vi "run_pharmaBotExp_v1.000.vi"(0 "data in":T12={"daq_ao 1"="Dev1/ao0", "daq_ai 1"="Dev1/ai0", "experiment day folder"=path "C:/multiBot/data/debug/testing", "Multiclamp init error"=0, "Multiclamp Handle Out"=10225184, "sampling rate (Hz)"=20000, "trial name"="t1"}, 1 "auto run?":bool, 3 "which manipulator":T13(ring), 4 "HEK/slice options":enum16{"slice", "HEK"}(ring), 5 "error in":errorcluster, 6 "Validate after Experiment":bool, 7 "common cluster":T9, 11 "individual controls in":T8, 13 "images":T3={"slice image"="remote image 00000000137F745C", "pipette template"="remote image 00000000137F7D5C", "found pipette"=refnum, "pipette mask for cell tracker"=refnum, "cell images ref"=refnum}) -> (10 "Cell Looks Good?":bool=TRUE, 12 "ValidationOutputCluster":T5(array[cluster]), 14 "ValidationResults":waveform(dbl)[][](array[waveform]), 15 "ValidationPos1":T6(array[ring]), 16 "Exp. Terminated":bool, 17 "ValidationPos2":T6(array[ring]), 18 "ValidationWaveform":waveform(dbl)[](array[waveform]), 19 "error out":errorcluster)   [LabVIEW 2019] (continued)
  in  "Gap Free Iclamp G":T33={"Which Position to use for Experiment"=enum."Don't Move", "Duration (s)"=10.0, "Valve 1 Position"=2, "Valve 2 Position"=2, "Replicates"=5.0, "Iholding (pA)"=200.0, "Valve 3 Position"=2, "valve 1 used now?"=TRUE, "valve 2 used now?"=FALSE, "valve 3 used now? "=FALSE, "Record During Solution Change?"=FALSE} {"Valve 3 Position" min=1 max=8; "Iholding (pA)" step=0.1; "Replicates" min=1.0 step=1.0; "Valve 2 Position" min=1 max=8; "Valve 1 Position" min=1 max=8; "Duration (s)" min=0.0 step=0.1}
  in  "PhaseH Experiment Option":string(combo)="Single Jump"
  in  "Experiment Selection H":T20(tab)
  in  "Single Jump H":T21={"Which Position to use for Experiment"=enum."Jumper Position B-A", "Start Position (N)"="Jumper Posistion B", "Jump Position (m)"="Jumper Posistion A", "Duration (s)"=5.0, "Delay (s)"=1.0, "Pulse Width (s)"=1.0, "Valve 1 Position"=2, "Valve 2 Position"=2, "Replicates"=1.0, "Vholding (mV)"=-60.0, "Valve 3 Position"=2, "valve 1 used now?"=TRUE, "valve 2 used now?"=FALSE, "valve 3 used now? "=FALSE, "protocol Preview"=[]} {"Valve 3 Position" min=1 max=8; "Vholding (mV)" step=0.1; "Replicates" min=1.0 step=1.0; "Valve 2 Position" min=1 max=8; "Valve 1 Position" min=1 max=8; "Pulse Width (s)" min=0.0 step=0.1; "Delay (s)" min=0.0 step=0.1; "Duration (s)" min=0.0 step=0.1}
  in  "Solution Change H":T22={"Which Position to use for Experiment"=enum."Jumper Safe Position", "Duration (s)"=60.0, "Delay (s)"=1.0, "Pulse Width (s)"=30.0, "Which Valve to Change?"=1, "Valve Jump Position"=3, "Replicates"=1.0, "Vholding (mV)"=-70.0, "valve 1 used now?"=TRUE, "valve 2 used now?"=FALSE, "valve 3 used now? "=FALSE, "Valve 1 Position"=2, "Valve 2 Position"=2, "Valve 3 Position"=2, "protocol Preview"=[]} {"Valve 3 Position" min=1 max=8; "Valve 2 Position" min=1 max=8; "Valve 1 Position" min=1 max=8; "Vholding (mV)" step=0.1; "Replicates" min=1.0 step=1.0; "Valve Jump Position" min=1 max=8 step=1; "Which Valve to Change?" min=1 max=8 step=1; "Pulse Width (s)" min=0.0 step=0.1; "Delay (s)" min=0.0 step=0.1; "Duration (s)" min=0.0 step=0.1}
  in  "Voltage Step H":T23={"Which Position to use for Experiment"=enum."Jumper Safe Position", "Duration (s)"=10.0, "Delay (s)"=1.0, "Step Width (s)"=0.1, "Voltage Start (mV)"=-60.0, "Voltage Step (mV)"=0.0, "Replicates"=1.0, "Voltage End (mV)"=40.0, "Number of Step"=20.0, "Vholding (mV)"=-60.0, "Valve 1 Position"=2, "Valve 2 Position"=2, "Valve 3 Position"=2, "valve 1 used now?"=TRUE, "valve 2 used now?"=FALSE, "valve 3 used now? "=FALSE, "Total Step Time (s)"=0.0, "Maintain Final Voltage until end?"=TRUE, "protocol Preview"=[]} {"Total Step Time (s)" min=0.0 step=0.1; "Valve 3 Position" min=1 max=8; "Valve 2 Position" min=1 max=8; "Valve 1 Position" min=1 max=8; "Vholding (mV)" step=0.1; "Number of Step" min=0.0 step=1.0; "Voltage End (mV)" step=0.1; "Replicates" min=1.0 step=1.0; "Voltage Step (mV)" step=0.1; "Voltage Start (mV)" step=0.1; "Step Width (s)" step=0.1; "Delay (s)" min=0.0 step=0.1; "Duration (s)" min=0.0 step=0.1}
  in  "Voltage Ramp H":T24={"Which Position to use for Experiment"=enum."Jumper Safe Position", "Duration (s)"=10.0, "Delay (s)"=1.0, "Ramp Slope (mV/s)"=0.0, "Voltage Start (mV)"=-60.0, "Replicates"=1.0, "Voltage End (mV)"=40.0, "Ramp Duration (s)"=5.0, "Vholding (mV)"=-60.0, "Valve 1 Position"=2, "Valve 2 Position"=2, "Valve 3 Position"=2, "valve 1 used now?"=TRUE, "valve 2 used now?"=FALSE, "valve 3 used now? "=FALSE, "Maintain Final Voltage until end?"=TRUE, "protocol Preview"=[]} {"Valve 3 Position" min=1 max=8; "Valve 2 Position" min=1 max=8; "Valve 1 Position" min=1 max=8; "Ramp Duration (s)" min=0.0 step=0.1; "Voltage End (mV)" step=0.1; "Replicates" min=1.0 step=1.0; "Voltage Start (mV)" step=0.1; "Ramp Slope (mV/s)" step=0.1; "Delay (s)" min=0.0 step=0.1; "Duration (s)" min=0.0 step=0.1}
  in  "Voltage Pulse H":T25={"Which Position to use for Experiment"=enum."Jumper Safe Position", "Duration (s)"=1.0, "Delay (s)"=0.2, "Pulse 2 (s)"=0.4, "Pulse 1 (mV)"=-80.0, "Replicates"=1.0, "Pulse 1 (s)"=0.2, "Pulse 2 (mV)"=-80.0, "Vholding (mV)"=-60.0, "Valve 1 Position"=2, "Valve 2 Position"=2, "Valve 3 Position"=2, "valve 1 used now?"=TRUE, "valve 2 used now?"=FALSE, "valve 3 used now? "=FALSE, "Maintain Final Voltage until end?"=TRUE, "delta Pulse 1 (mV)"=0.0, "delta Pulse 2 (mV)"=5.0, "Sweeps"=24.0, "Final Pulse 1 (mV)"=0.0, "Final Pulse 2 (mV)"=0.0, "protocol Preview"=[]} {"Final Pulse 2 (mV)" step=0.1; "Final Pulse 1 (mV)" step=0.1; "Sweeps" min=1.0 step=1.0; "delta Pulse 2 (mV)" step=0.1; "delta Pulse 1 (mV)" step=0.1; "Valve 3 Position" min=1 max=8; "Valve 2 Position" min=1 max=8; "Valve 1 Position" min=1 max=8; "Vholding (mV)" step=0.1; "Pulse 2 (mV)" step=0.1; "Pulse 1 (s)" min=0.0 step=0.1; "Replicates" min=1.0 step=1.0; "Pulse 1 (mV)" step=0.1; "Pulse 2 (s)" min=0.0 step=0.1; "Delay (s)" min=0.0 step=0.1; "Duration (s)" min=0.0 step=0.1}
  in  "Jump Train H":T26={"Which Position to use for Experiment"=enum."Jumper Safe Position", "Start Position (N)"="", "Jump Position (m)"="", "Duration (s)"=20.0, "Delay (s)"=1.0, "Pulse Width (s)"=1.0, "Valve 1 Position"=1, "Valve 2 Position"=1, "Replicates"=1.0, "Pulse Period (s)"=2.0, "Vholding (mV)"=-60.0, "Number of Pulses"=5.0, "valve 1 used now?"=TRUE, "valve 2 used now?"=FALSE, "valve 3 used now? "=FALSE, "Valve 3 Position"=1, "protocol Preview"=[]} {"Valve 3 Position" min=1 max=8; "Number of Pulses" min=0.0 step=1.0; "Vholding (mV)" step=0.1; "Pulse Period (s)" min=0.0 step=0.1; "Replicates" min=1.0 step=1.0; "Valve 2 Position" min=1 max=8; "Valve 1 Position" min=1 max=8; "Pulse Width (s)" min=0.0 step=0.1; "Delay (s)" min=0.0 step=0.1; "Duration (s)" min=0.0 step=0.1}
  in  "Paired Pulse H":T27={"Which Position to use for Experiment"=enum."Jumper Safe Position", "Start Position (N)"="", "Jump Position (m)"="", "Duration (s)"=10.0, "Delay (s)"=1.0, "Pulse Width (s)"=1.0, "Replicates"=1.0, "Pulse Delay (s)"=1.0, "Pulse Delta Delay (s)"=0.5, "Vholding (mV)"=-60.0, "Valve 1 Position"=1, "Valve 2 Position"=1, "valve 1 used now?"=TRUE, "valve 2 used now?"=FALSE, "valve 3 used now? "=FALSE, "Valve 3 Position"=1, "protocol Preview"=[]} {"Valve 3 Position" min=1 max=8; "Valve 2 Position" min=1 max=8; "Valve 1 Position" min=1 max=8; "Vholding (mV)" step=0.1; "Pulse Delta Delay (s)" min=0.0 step=0.1; "Pulse Delay (s)" min=0.0 step=0.1; "Replicates" min=1.0 step=1.0; "Pulse Width (s)" min=0.0 step=0.1; "Delay (s)" min=0.0 step=0.1; "Duration (s)" min=0.0 step=0.1}
  in  "Single Manip Jump H":T28={"Start Position (N)"=enum."Jumper Position B", "Duration (s)"=8.0, "Delay (s)"=0.5, "Pulse Width (s)"=1.0, "Valve 1 Position"=2, "Valve 2 Position"=2, "Replicates"=10.0, "Jump Position (m)"=enum."Jumper Position A", "Vholding (mV)"=-60.0, "Valve 3 Position"=2, "valve 1 used now?"=TRUE, "valve 2 used now?"=FALSE, "valve 3 used now? "=FALSE, "protocol Preview"=[]} {"Valve 3 Position" min=1 max=8; "Vholding (mV)" step=0.1; "Replicates" min=1.0 step=1.0; "Valve 2 Position" min=1 max=8; "Valve 1 Position" min=1 max=8; "Pulse Width (s)" min=0.0 step=0.1; "Delay (s)" min=0.0 step=0.1; "Duration (s)" min=0.0 step=0.1}
  in  "Gap Free H":T29={"Which Position to use for Experiment"=enum."Don't Move", "Duration (s)"=120.0, "Valve 1 Position"=1, "Valve 2 Position"=1, "Replicates"=2.0, "Vholding (mV)"=-60.0, "Valve 3 Position"=1, "valve 1 used now?"=TRUE, "valve 2 used now?"=FALSE, "valve 3 used now? "=FALSE, "Record During Solution Change?"=TRUE} {"Valve 3 Position" min=1 max=8; "Vholding (mV)" step=0.1; "Replicates" min=1.0 step=1.0; "Valve 2 Position" min=1 max=8; "Valve 1 Position" min=1 max=8; "Duration (s)" min=0.0 step=0.1}
  in  "Multi Manip Jump H":T30={"Start Position (N)"=enum."Jumper Position C", "Duration (s)"=20.0, "Delay (s)"=2.0, "Valve 1 Position"=2, "Valve 2 Position"=2, "Replicates"=5.0, "Vholding (mV)"=-60.0, "Valve 3 Position"=2, "valve 1 used now?"=TRUE, "valve 2 used now?"=FALSE, "valve 3 used now? "=FALSE, "Jump Position Array"=[enum."Jumper Position B", enum."Jumper Position A", enum."Jumper Position B", enum."Jumper Position C"], "Position Dwell Time (s)"=[2.0, 4.0, 4.0, 4.0], "protocol Preview"=[]} {"Position Dwell Time (s)" min=0.0 step=0.1; "Vholding (mV)" step=0.1; "Replicates" min=1.0 step=1.0; "Valve 2 Position" min=1 max=8; "Delay (s)" min=0.0 step=0.1; "Duration (s)" min=0.0 step=0.1}
  in  "Current Pulse H":T31={"Which Position to use for Experiment"=enum."Jumper Safe Position", "Duration (s)"=1.0, "Delay (s)"=0.2, "Pulse 2 (s)"=0.4, "Pulse 1 (pA)"=-400.0, "Replicates"=1.0, "Pulse 1 (s)"=0.6, "Pulse 2 (pA)"=-80.0, "Iholding (pA)"=0.0, "Valve 1 Position"=2, "Valve 2 Position"=2, "Valve 3 Position"=2, "valve 1 used now?"=TRUE, "valve 2 used now?"=FALSE, "valve 3 used now? "=FALSE, "Maintain Final Voltage until end?"=FALSE, "delta Pulse 1 (pA)"=50.0, "delta Pulse 2 (pA)"=5.0, "Sweeps"=24.0, "Final Pulse 1 (pA)"=0.0, "Final Pulse 2 (pA)"=0.0, "protocol Preview"=[]} {"Final Pulse 2 (pA)" step=0.1; "Final Pulse 1 (pA)" step=0.1; "Sweeps" min=1.0 step=1.0; "delta Pulse 2 (pA)" step=0.1; "delta Pulse 1 (pA)" step=0.1; "Valve 3 Position" min=1 max=8; "Valve 2 Position" min=1 max=8; "Valve 1 Position" min=1 max=8; "Iholding (pA)" step=0.1; "Pulse 2 (pA)" step=0.1; "Pulse 1 (s)" min=0.0 step=0.1; "Replicates" min=1.0 step=1.0; "Pulse 1 (pA)" step=0.1; "Pulse 2 (s)" min=0.0 step=0.1; "Delay (s)" min=0.0 step=0.1; "Duration (s)" min=0.0 step=0.1}
  in  "Current Ramp H":T32={"Which Position to use for Experiment"=enum."Jumper Safe Position", "Duration (s)"=10.0, "Delay (s)"=1.0, "Ramp Slope (pA/s)"=0.0, "Current Start (pA)"=-200.0, "Replicates"=1.0, "Current End (pA)"=500.0, "Ramp Duration (s)"=5.0, "Iholding (pA)"=0.0, "Valve 1 Position"=2, "Valve 2 Position"=2, "Valve 3 Position"=2, "valve 1 used now?"=TRUE, "valve 2 used now?"=FALSE, "valve 3 used now? "=FALSE, "Maintain Final Voltage until end?"=FALSE, "protocol Preview"=[]} {"Valve 3 Position" min=1 max=8; "Valve 2 Position" min=1 max=8; "Valve 1 Position" min=1 max=8; "Ramp Duration (s)" min=0.0 step=0.1; "Current End (pA)" step=0.1; "Replicates" min=1.0 step=1.0; "Current Start (pA)" step=0.1; "Ramp Slope (pA/s)" step=0.1; "Delay (s)" min=0.0 step=0.1; "Duration (s)" min=0.0 step=0.1}
  in  "Gap Free Iclamp H":T33={"Which Position to use for Experiment"=enum."Don't Move", "Duration (s)"=10.0, "Valve 1 Position"=2, "Valve 2 Position"=2, "Replicates"=5.0, "Iholding (pA)"=200.0, "Valve 3 Position"=2, "valve 1 used now?"=TRUE, "valve 2 used now?"=FALSE, "valve 3 used now? "=FALSE, "Record During Solution Change?"=FALSE} {"Valve 3 Position" min=1 max=8; "Iholding (pA)" step=0.1; "Replicates" min=1.0 step=1.0; "Valve 2 Position" min=1 max=8; "Valve 1 Position" min=1 max=8; "Duration (s)" min=0.0 step=0.1}
  in  "PhaseI Experiment Option":string(combo)="Single Manip Jump"
  in  "Experiment Selection I":T20(tab)=enum."Single Manip Jump"
  in  "Single Jump I":T21={"Which Position to use for Experiment"=enum."Jumper Position B-A", "Start Position (N)"="Jumper Posistion B", "Jump Position (m)"="Jumper Posistion A", "Duration (s)"=5.0, "Delay (s)"=1.0, "Pulse Width (s)"=1.0, "Valve 1 Position"=2, "Valve 2 Position"=2, "Replicates"=10.0, "Vholding (mV)"=-60.0, "Valve 3 Position"=2, "valve 1 used now?"=TRUE, "valve 2 used now?"=FALSE, "valve 3 used now? "=FALSE, "protocol Preview"=[]} {"Valve 3 Position" min=1 max=8; "Vholding (mV)" step=0.1; "Replicates" min=1.0 step=1.0; "Valve 2 Position" min=1 max=8; "Valve 1 Position" min=1 max=8; "Pulse Width (s)" min=0.0 step=0.1; "Delay (s)" min=0.0 step=0.1; "Duration (s)" min=0.0 step=0.1}
  in  "Solution Change I":T22={"Which Position to use for Experiment"=enum."Jumper Safe Position", "Duration (s)"=60.0, "Delay (s)"=1.0, "Pulse Width (s)"=30.0, "Which Valve to Change?"=1, "Valve Jump Position"=3, "Replicates"=1.0, "Vholding (mV)"=-70.0, "valve 1 used now?"=TRUE, "valve 2 used now?"=FALSE, "valve 3 used now? "=FALSE, "Valve 1 Position"=2, "Valve 2 Position"=2, "Valve 3 Position"=2, "protocol Preview"=[]} {"Valve 3 Position" min=1 max=8; "Valve 2 Position" min=1 max=8; "Valve 1 Position" min=1 max=8; "Vholding (mV)" step=0.1; "Replicates" min=1.0 step=1.0; "Valve Jump Position" min=1 max=8 step=1; "Which Valve to Change?" min=1 max=8 step=1; "Pulse Width (s)" min=0.0 step=0.1; "Delay (s)" min=0.0 step=0.1; "Duration (s)" min=0.0 step=0.1}
  in  "Voltage Step I":T23={"Which Position to use for Experiment"=enum."Jumper Safe Position", "Duration (s)"=10.0, "Delay (s)"=1.0, "Step Width (s)"=0.1, "Voltage Start (mV)"=-60.0, "Voltage Step (mV)"=0.0, "Replicates"=1.0, "Voltage End (mV)"=40.0, "Number of Step"=20.0, "Vholding (mV)"=-60.0, "Valve 1 Position"=2, "Valve 2 Position"=2, "Valve 3 Position"=2, "valve 1 used now?"=TRUE, "valve 2 used now?"=FALSE, "valve 3 used now? "=FALSE, "Total Step Time (s)"=0.0, "Maintain Final Voltage until end?"=TRUE, "protocol Preview"=[]} {"Total Step Time (s)" min=0.0 step=0.1; "Valve 3 Position" min=1 max=8; "Valve 2 Position" min=1 max=8; "Valve 1 Position" min=1 max=8; "Vholding (mV)" step=0.1; "Number of Step" min=0.0 step=1.0; "Voltage End (mV)" step=0.1; "Replicates" min=1.0 step=1.0; "Voltage Step (mV)" step=0.1; "Voltage Start (mV)" step=0.1; "Step Width (s)" step=0.1; "Delay (s)" min=0.0 step=0.1; "Duration (s)" min=0.0 step=0.1}
  in  "Voltage Ramp I":T24={"Which Position to use for Experiment"=enum."Jumper Safe Position", "Duration (s)"=10.0, "Delay (s)"=1.0, "Ramp Slope (mV/s)"=0.0, "Voltage Start (mV)"=-60.0, "Replicates"=1.0, "Voltage End (mV)"=40.0, "Ramp Duration (s)"=5.0, "Vholding (mV)"=-60.0, "Valve 1 Position"=2, "Valve 2 Position"=2, "Valve 3 Position"=2, "valve 1 used now?"=TRUE, "valve 2 used now?"=FALSE, "valve 3 used now? "=FALSE, "Maintain Final Voltage until end?"=TRUE, "protocol Preview"=[]} {"Valve 3 Position" min=1 max=8; "Valve 2 Position" min=1 max=8; "Valve 1 Position" min=1 max=8; "Ramp Duration (s)" min=0.0 step=0.1; "Voltage End (mV)" step=0.1; "Replicates" min=1.0 step=1.0; "Voltage Start (mV)" step=0.1; "Ramp Slope (mV/s)" step=0.1; "Delay (s)" min=0.0 step=0.1; "Duration (s)" min=0.0 step=0.1}
  in  "Voltage Pulse I":T25={"Which Position to use for Experiment"=enum."Jumper Safe Position", "Duration (s)"=1.0, "Delay (s)"=0.2, "Pulse 2 (s)"=0.4, "Pulse 1 (mV)"=-80.0, "Replicates"=1.0, "Pulse 1 (s)"=0.2, "Pulse 2 (mV)"=-80.0, "Vholding (mV)"=-60.0, "Valve 1 Position"=2, "Valve 2 Position"=2, "Valve 3 Position"=2, "valve 1 used now?"=TRUE, "valve 2 used now?"=FALSE, "valve 3 used now? "=FALSE, "Maintain Final Voltage until end?"=TRUE, "delta Pulse 1 (mV)"=0.0, "delta Pulse 2 (mV)"=5.0, "Sweeps"=24.0, "Final Pulse 1 (mV)"=0.0, "Final Pulse 2 (mV)"=0.0, "protocol Preview"=[]} {"Final Pulse 2 (mV)" step=0.1; "Final Pulse 1 (mV)" step=0.1; "Sweeps" min=1.0 step=1.0; "delta Pulse 2 (mV)" step=0.1; "delta Pulse 1 (mV)" step=0.1; "Valve 3 Position" min=1 max=8; "Valve 2 Position" min=1 max=8; "Valve 1 Position" min=1 max=8; "Vholding (mV)" step=0.1; "Pulse 2 (mV)" step=0.1; "Pulse 1 (s)" min=0.0 step=0.1; "Replicates" min=1.0 step=1.0; "Pulse 1 (mV)" step=0.1; "Pulse 2 (s)" min=0.0 step=0.1; "Delay (s)" min=0.0 step=0.1; "Duration (s)" min=0.0 step=0.1}
  in  "Jump Train I":T26={"Which Position to use for Experiment"=enum."Jumper Safe Position", "Start Position (N)"="", "Jump Position (m)"="", "Duration (s)"=20.0, "Delay (s)"=1.0, "Pulse Width (s)"=1.0, "Valve 1 Position"=1, "Valve 2 Position"=1, "Replicates"=1.0, "Pulse Period (s)"=2.0, "Vholding (mV)"=-60.0, "Number of Pulses"=5.0, "valve 1 used now?"=TRUE, "valve 2 used now?"=FALSE, "valve 3 used now? "=FALSE, "Valve 3 Position"=1, "protocol Preview"=[]} {"Valve 3 Position" min=1 max=8; "Number of Pulses" min=0.0 step=1.0; "Vholding (mV)" step=0.1; "Pulse Period (s)" min=0.0 step=0.1; "Replicates" min=1.0 step=1.0; "Valve 2 Position" min=1 max=8; "Valve 1 Position" min=1 max=8; "Pulse Width (s)" min=0.0 step=0.1; "Delay (s)" min=0.0 step=0.1; "Duration (s)" min=0.0 step=0.1}
  in  "Paired Pulse I":T27={"Which Position to use for Experiment"=enum."Jumper Safe Position", "Start Position (N)"="", "Jump Position (m)"="", "Duration (s)"=10.0, "Delay (s)"=1.0, "Pulse Width (s)"=1.0, "Replicates"=1.0, "Pulse Delay (s)"=1.0, "Pulse Delta Delay (s)"=0.5, "Vholding (mV)"=-60.0, "Valve 1 Position"=1, "Valve 2 Position"=1, "valve 1 used now?"=TRUE, "valve 2 used now?"=FALSE, "valve 3 used now? "=FALSE, "Valve 3 Position"=1, "protocol Preview"=[]} {"Valve 3 Position" min=1 max=8; "Valve 2 Position" min=1 max=8; "Valve 1 Position" min=1 max=8; "Vholding (mV)" step=0.1; "Pulse Delta Delay (s)" min=0.0 step=0.1; "Pulse Delay (s)" min=0.0 step=0.1; "Replicates" min=1.0 step=1.0; "Pulse Width (s)" min=0.0 step=0.1; "Delay (s)" min=0.0 step=0.1; "Duration (s)" min=0.0 step=0.1}
  in  "Single Manip Jump I":T28={"Start Position (N)"=enum."Jumper Position B", "Duration (s)"=8.0, "Delay (s)"=0.5, "Pulse Width (s)"=1.0, "Valve 1 Position"=2, "Valve 2 Position"=2, "Replicates"=1.0, "Jump Position (m)"=enum."Jumper Position A", "Vholding (mV)"=-60.0, "Valve 3 Position"=2, "valve 1 used now?"=TRUE, "valve 2 used now?"=FALSE, "valve 3 used now? "=FALSE, "protocol Preview"=[]} {"Valve 3 Position" min=1 max=8; "Vholding (mV)" step=0.1; "Replicates" min=1.0 step=1.0; "Valve 2 Position" min=1 max=8; "Valve 1 Position" min=1 max=8; "Pulse Width (s)" min=0.0 step=0.1; "Delay (s)" min=0.0 step=0.1; "Duration (s)" min=0.0 step=0.1}
  in  "Gap Free I":T29={"Which Position to use for Experiment"=enum."Jumper Position B", "Duration (s)"=10.0, "Valve 1 Position"=2, "Valve 2 Position"=2, "Replicates"=5.0, "Vholding (mV)"=-60.0, "Valve 3 Position"=2, "valve 1 used now?"=TRUE, "valve 2 used now?"=FALSE, "valve 3 used now? "=FALSE, "Record During Solution Change?"=FALSE} {"Valve 3 Position" min=1 max=8; "Vholding (mV)" step=0.1; "Replicates" min=1.0 step=1.0; "Valve 2 Position" min=1 max=8; "Valve 1 Position" min=1 max=8; "Duration (s)" min=0.0 step=0.1}
  in  "Multi Manip Jump I":T30={"Start Position (N)"=enum."Jumper Position C", "Duration (s)"=20.0, "Delay (s)"=2.0, "Valve 1 Position"=2, "Valve 2 Position"=2, "Replicates"=5.0, "Vholding (mV)"=-60.0, "Valve 3 Position"=2, "valve 1 used now?"=TRUE, "valve 2 used now?"=FALSE, "valve 3 used now? "=FALSE, "Jump Position Array"=[enum."Jumper Position B", enum."Jumper Position A", enum."Jumper Position B", enum."Jumper Position C"], "Position Dwell Time (s)"=[2.0, 4.0, 4.0, 4.0], "protocol Preview"=[]} {"Position Dwell Time (s)" min=0.0 step=0.1; "Vholding (mV)" step=0.1; "Replicates" min=1.0 step=1.0; "Valve 2 Position" min=1 max=8; "Delay (s)" min=0.0 step=0.1; "Duration (s)" min=0.0 step=0.1}
  in  "Current Pulse I":T31={"Which Position to use for Experiment"=enum."Jumper Safe Position", "Duration (s)"=1.0, "Delay (s)"=0.2, "Pulse 2 (s)"=0.4, "Pulse 1 (pA)"=-400.0, "Replicates"=1.0, "Pulse 1 (s)"=0.6, "Pulse 2 (pA)"=-80.0, "Iholding (pA)"=0.0, "Valve 1 Position"=2, "Valve 2 Position"=2, "Valve 3 Position"=2, "valve 1 used now?"=TRUE, "valve 2 used now?"=FALSE, "valve 3 used now? "=FALSE, "Maintain Final Voltage until end?"=FALSE, "delta Pulse 1 (pA)"=50.0, "delta Pulse 2 (pA)"=5.0, "Sweeps"=24.0, "Final Pulse 1 (pA)"=0.0, "Final Pulse 2 (pA)"=0.0, "protocol Preview"=[]} {"Final Pulse 2 (pA)" step=0.1; "Final Pulse 1 (pA)" step=0.1; "Sweeps" min=1.0 step=1.0; "delta Pulse 2 (pA)" step=0.1; "delta Pulse 1 (pA)" step=0.1; "Valve 3 Position" min=1 max=8; "Valve 2 Position" min=1 max=8; "Valve 1 Position" min=1 max=8; "Iholding (pA)" step=0.1; "Pulse 2 (pA)" step=0.1; "Pulse 1 (s)" min=0.0 step=0.1; "Replicates" min=1.0 step=1.0; "Pulse 1 (pA)" step=0.1; "Pulse 2 (s)" min=0.0 step=0.1; "Delay (s)" min=0.0 step=0.1; "Duration (s)" min=0.0 step=0.1}
  in  "Current Ramp I":T32={"Which Position to use for Experiment"=enum."Jumper Safe Position", "Duration (s)"=10.0, "Delay (s)"=1.0, "Ramp Slope (pA/s)"=0.0, "Current Start (pA)"=-200.0, "Replicates"=1.0, "Current End (pA)"=500.0, "Ramp Duration (s)"=5.0, "Iholding (pA)"=0.0, "Valve 1 Position"=2, "Valve 2 Position"=2, "Valve 3 Position"=2, "valve 1 used now?"=TRUE, "valve 2 used now?"=FALSE, "valve 3 used now? "=FALSE, "Maintain Final Voltage until end?"=FALSE, "protocol Preview"=[]} {"Valve 3 Position" min=1 max=8; "Valve 2 Position" min=1 max=8; "Valve 1 Position" min=1 max=8; "Ramp Duration (s)" min=0.0 step=0.1; "Current End (pA)" step=0.1; "Replicates" min=1.0 step=1.0; "Current Start (pA)" step=0.1; "Ramp Slope (pA/s)" step=0.1; "Delay (s)" min=0.0 step=0.1; "Duration (s)" min=0.0 step=0.1}
  in  "Gap Free Iclamp I":T33={"Which Position to use for Experiment"=enum."Don't Move", "Duration (s)"=10.0, "Valve 1 Position"=2, "Valve 2 Position"=2, "Replicates"=5.0, "Iholding (pA)"=200.0, "Valve 3 Position"=2, "valve 1 used now?"=TRUE, "valve 2 used now?"=FALSE, "valve 3 used now? "=FALSE, "Record During Solution Change?"=FALSE} {"Valve 3 Position" min=1 max=8; "Iholding (pA)" step=0.1; "Replicates" min=1.0 step=1.0; "Valve 2 Position" min=1 max=8; "Valve 1 Position" min=1 max=8; "Duration (s)" min=0.0 step=0.1}
  in  "PhaseJ Experiment Option":string(combo)="Multi M. Jump"
  in  "Experiment Selection J":T20(tab)=enum."Multi M. Jump"
  in  "Single Jump J":T21={"Which Position to use for Experiment"=enum."Jumper Position B-A", "Start Position (N)"="Jumper Posistion B", "Jump Position (m)"="Jumper Posistion A", "Duration (s)"=5.0, "Delay (s)"=1.0, "Pulse Width (s)"=1.0, "Valve 1 Position"=2, "Valve 2 Position"=2, "Replicates"=10.0, "Vholding (mV)"=-60.0, "Valve 3 Position"=2, "valve 1 used now?"=TRUE, "valve 2 used now?"=FALSE, "valve 3 used now? "=FALSE, "protocol Preview"=[]} {"Valve 3 Position" min=1 max=8; "Vholding (mV)" step=0.1; "Replicates" min=1.0 step=1.0; "Valve 2 Position" min=1 max=8; "Valve 1 Position" min=1 max=8; "Pulse Width (s)" min=0.0 step=0.1; "Delay (s)" min=0.0 step=0.1; "Duration (s)" min=0.0 step=0.1}
  in  "Solution Change J":T22={"Which Position to use for Experiment"=enum."Jumper Safe Position", "Duration (s)"=60.0, "Delay (s)"=1.0, "Pulse Width (s)"=30.0, "Which Valve to Change?"=1, "Valve Jump Position"=3, "Replicates"=1.0, "Vholding (mV)"=-70.0, "valve 1 used now?"=TRUE, "valve 2 used now?"=FALSE, "valve 3 used now? "=FALSE, "Valve 1 Position"=2, "Valve 2 Position"=2, "Valve 3 Position"=2, "protocol Preview"=[]} {"Valve 3 Position" min=1 max=8; "Valve 2 Position" min=1 max=8; "Valve 1 Position" min=1 max=8; "Vholding (mV)" step=0.1; "Replicates" min=1.0 step=1.0; "Valve Jump Position" min=1 max=8 step=1; "Which Valve to Change?" min=1 max=8 step=1; "Pulse Width (s)" min=0.0 step=0.1; "Delay (s)" min=0.0 step=0.1; "Duration (s)" min=0.0 step=0.1}
  in  "Voltage Step J":T23={"Which Position to use for Experiment"=enum."Jumper Safe Position", "Duration (s)"=10.0, "Delay (s)"=1.0, "Step Width (s)"=0.1, "Voltage Start (mV)"=-60.0, "Voltage Step (mV)"=0.0, "Replicates"=1.0, "Voltage End (mV)"=40.0, "Number of Step"=20.0, "Vholding (mV)"=-60.0, "Valve 1 Position"=2, "Valve 2 Position"=2, "Valve 3 Position"=2, "valve 1 used now?"=TRUE, "valve 2 used now?"=FALSE, "valve 3 used now? "=FALSE, "Total Step Time (s)"=0.0, "Maintain Final Voltage until end?"=TRUE, "protocol Preview"=[]} {"Total Step Time (s)" min=0.0 step=0.1; "Valve 3 Position" min=1 max=8; "Valve 2 Position" min=1 max=8; "Valve 1 Position" min=1 max=8; "Vholding (mV)" step=0.1; "Number of Step" min=0.0 step=1.0; "Voltage End (mV)" step=0.1; "Replicates" min=1.0 step=1.0; "Voltage Step (mV)" step=0.1; "Voltage Start (mV)" step=0.1; "Step Width (s)" step=0.1; "Delay (s)" min=0.0 step=0.1; "Duration (s)" min=0.0 step=0.1}
  in  "Voltage Ramp J":T24={"Which Position to use for Experiment"=enum."Jumper Safe Position", "Duration (s)"=10.0, "Delay (s)"=1.0, "Ramp Slope (mV/s)"=0.0, "Voltage Start (mV)"=-60.0, "Replicates"=1.0, "Voltage End (mV)"=40.0, "Ramp Duration (s)"=5.0, "Vholding (mV)"=-60.0, "Valve 1 Position"=2, "Valve 2 Position"=2, "Valve 3 Position"=2, "valve 1 used now?"=TRUE, "valve 2 used now?"=FALSE, "valve 3 used now? "=FALSE, "Maintain Final Voltage until end?"=TRUE, "protocol Preview"=[]} {"Valve 3 Position" min=1 max=8; "Valve 2 Position" min=1 max=8; "Valve 1 Position" min=1 max=8; "Ramp Duration (s)" min=0.0 step=0.1; "Voltage End (mV)" step=0.1; "Replicates" min=1.0 step=1.0; "Voltage Start (mV)" step=0.1; "Ramp Slope (mV/s)" step=0.1; "Delay (s)" min=0.0 step=0.1; "Duration (s)" min=0.0 step=0.1}
  in  "Voltage Pulse J":T25={"Which Position to use for Experiment"=enum."Jumper Safe Position", "Duration (s)"=1.0, "Delay (s)"=0.2, "Pulse 2 (s)"=0.4, "Pulse 1 (mV)"=-80.0, "Replicates"=1.0, "Pulse 1 (s)"=0.2, "Pulse 2 (mV)"=-80.0, "Vholding (mV)"=-60.0, "Valve 1 Position"=2, "Valve 2 Position"=2, "Valve 3 Position"=2, "valve 1 used now?"=TRUE, "valve 2 used now?"=FALSE, "valve 3 used now? "=FALSE, "Maintain Final Voltage until end?"=TRUE, "delta Pulse 1 (mV)"=0.0, "delta Pulse 2 (mV)"=5.0, "Sweeps"=24.0, "Final Pulse 1 (mV)"=0.0, "Final Pulse 2 (mV)"=0.0, "protocol Preview"=[]} {"Final Pulse 2 (mV)" step=0.1; "Final Pulse 1 (mV)" step=0.1; "Sweeps" min=1.0 step=1.0; "delta Pulse 2 (mV)" step=0.1; "delta Pulse 1 (mV)" step=0.1; "Valve 3 Position" min=1 max=8; "Valve 2 Position" min=1 max=8; "Valve 1 Position" min=1 max=8; "Vholding (mV)" step=0.1; "Pulse 2 (mV)" step=0.1; "Pulse 1 (s)" min=0.0 step=0.1; "Replicates" min=1.0 step=1.0; "Pulse 1 (mV)" step=0.1; "Pulse 2 (s)" min=0.0 step=0.1; "Delay (s)" min=0.0 step=0.1; "Duration (s)" min=0.0 step=0.1}
  in  "Jump Train J":T26={"Which Position to use for Experiment"=enum."Jumper Safe Position", "Start Position (N)"="", "Jump Position (m)"="", "Duration (s)"=20.0, "Delay (s)"=1.0, "Pulse Width (s)"=1.0, "Valve 1 Position"=1, "Valve 2 Position"=1, "Replicates"=1.0, "Pulse Period (s)"=2.0, "Vholding (mV)"=-60.0, "Number of Pulses"=5.0, "valve 1 used now?"=TRUE, "valve 2 used now?"=FALSE, "valve 3 used now? "=FALSE, "Valve 3 Position"=1, "protocol Preview"=[]} {"Valve 3 Position" min=1 max=8; "Number of Pulses" min=0.0 step=1.0; "Vholding (mV)" step=0.1; "Pulse Period (s)" min=0.0 step=0.1; "Replicates" min=1.0 step=1.0; "Valve 2 Position" min=1 max=8; "Valve 1 Position" min=1 max=8; "Pulse Width (s)" min=0.0 step=0.1; "Delay (s)" min=0.0 step=0.1; "Duration (s)" min=0.0 step=0.1}
  in  "Paired Pulse J":T27={"Which Position to use for Experiment"=enum."Jumper Safe Position", "Start Position (N)"="", "Jump Position (m)"="", "Duration (s)"=10.0, "Delay (s)"=1.0, "Pulse Width (s)"=1.0, "Replicates"=1.0, "Pulse Delay (s)"=1.0, "Pulse Delta Delay (s)"=0.5, "Vholding (mV)"=-60.0, "Valve 1 Position"=1, "Valve 2 Position"=1, "valve 1 used now?"=TRUE, "valve 2 used now?"=FALSE, "valve 3 used now? "=FALSE, "Valve 3 Position"=1, "protocol Preview"=[]} {"Valve 3 Position" min=1 max=8; "Valve 2 Position" min=1 max=8; "Valve 1 Position" min=1 max=8; "Vholding (mV)" step=0.1; "Pulse Delta Delay (s)" min=0.0 step=0.1; "Pulse Delay (s)" min=0.0 step=0.1; "Replicates" min=1.0 step=1.0; "Pulse Width (s)" min=0.0 step=0.1; "Delay (s)" min=0.0 step=0.1; "Duration (s)" min=0.0 step=0.1}
  in  "Single Manip Jump J":T28={"Start Position (N)"=enum."Jumper Position B", "Duration (s)"=8.0, "Delay (s)"=0.5, "Pulse Width (s)"=1.0, "Valve 1 Position"=2, "Valve 2 Position"=2, "Replicates"=10.0, "Jump Position (m)"=enum."Jumper Position A", "Vholding (mV)"=-60.0, "Valve 3 Position"=2, "valve 1 used now?"=TRUE, "valve 2 used now?"=FALSE, "valve 3 used now? "=FALSE, "protocol Preview"=[]} {"Valve 3 Position" min=1 max=8; "Vholding (mV)" step=0.1; "Replicates" min=1.0 step=1.0; "Valve 2 Position" min=1 max=8; "Valve 1 Position" min=1 max=8; "Pulse Width (s)" min=0.0 step=0.1; "Delay (s)" min=0.0 step=0.1; "Duration (s)" min=0.0 step=0.1}
  in  "Gap Free J":T29={"Which Position to use for Experiment"=enum."Jumper Position B", "Duration (s)"=10.0, "Valve 1 Position"=2, "Valve 2 Position"=2, "Replicates"=5.0, "Vholding (mV)"=-60.0, "Valve 3 Position"=2, "valve 1 used now?"=TRUE, "valve 2 used now?"=FALSE, "valve 3 used now? "=FALSE, "Record During Solution Change?"=FALSE} {"Valve 3 Position" min=1 max=8; "Vholding (mV)" step=0.1; "Replicates" min=1.0 step=1.0; "Valve 2 Position" min=1 max=8; "Valve 1 Position" min=1 max=8; "Duration (s)" min=0.0 step=0.1}
  in  "Multi Manip Jump J":T30={"Start Position (N)"=enum."Jumper Position C", "Duration (s)"=20.0, "Delay (s)"=2.0, "Valve 1 Position"=2, "Valve 2 Position"=2, "Replicates"=1.0, "Vholding (mV)"=-60.0, "Valve 3 Position"=2, "valve 1 used now?"=TRUE, "valve 2 used now?"=FALSE, "valve 3 used now? "=FALSE, "Jump Position Array"=[enum."Jumper Position B", enum."Jumper Position A", enum."Jumper Position B", enum."Jumper Position C"], "Position Dwell Time (s)"=[2.0, 4.0, 4.0, 4.0], "protocol Preview"=[]} {"Position Dwell Time (s)" min=0.0 step=0.1; "Vholding (mV)" step=0.1; "Replicates" min=1.0 step=1.0; "Valve 2 Position" min=1 max=8; "Delay (s)" min=0.0 step=0.1; "Duration (s)" min=0.0 step=0.1}
  in  "Current Pulse J":T31={"Which Position to use for Experiment"=enum."Jumper Safe Position", "Duration (s)"=1.0, "Delay (s)"=0.2, "Pulse 2 (s)"=0.4, "Pulse 1 (pA)"=-400.0, "Replicates"=1.0, "Pulse 1 (s)"=0.6, "Pulse 2 (pA)"=-80.0, "Iholding (pA)"=0.0, "Valve 1 Position"=2, "Valve 2 Position"=2, "Valve 3 Position"=2, "valve 1 used now?"=TRUE, "valve 2 used now?"=FALSE, "valve 3 used now? "=FALSE, "Maintain Final Voltage until end?"=FALSE, "delta Pulse 1 (pA)"=50.0, "delta Pulse 2 (pA)"=5.0, "Sweeps"=24.0, "Final Pulse 1 (pA)"=0.0, "Final Pulse 2 (pA)"=0.0, "protocol Preview"=[]} {"Final Pulse 2 (pA)" step=0.1; "Final Pulse 1 (pA)" step=0.1; "Sweeps" min=1.0 step=1.0; "delta Pulse 2 (pA)" step=0.1; "delta Pulse 1 (pA)" step=0.1; "Valve 3 Position" min=1 max=8; "Valve 2 Position" min=1 max=8; "Valve 1 Position" min=1 max=8; "Iholding (pA)" step=0.1; "Pulse 2 (pA)" step=0.1; "Pulse 1 (s)" min=0.0 step=0.1; "Replicates" min=1.0 step=1.0; "Pulse 1 (pA)" step=0.1; "Pulse 2 (s)" min=0.0 step=0.1; "Delay (s)" min=0.0 step=0.1; "Duration (s)" min=0.0 step=0.1}
  in  "Current Ramp J":T32={"Which Position to use for Experiment"=enum."Jumper Safe Position", "Duration (s)"=10.0, "Delay (s)"=1.0, "Ramp Slope (pA/s)"=0.0, "Current Start (pA)"=-200.0, "Replicates"=1.0, "Current End (pA)"=500.0, "Ramp Duration (s)"=5.0, "Iholding (pA)"=0.0, "Valve 1 Position"=2, "Valve 2 Position"=2, "Valve 3 Position"=2, "valve 1 used now?"=TRUE, "valve 2 used now?"=FALSE, "valve 3 used now? "=FALSE, "Maintain Final Voltage until end?"=FALSE, "protocol Preview"=[]} {"Valve 3 Position" min=1 max=8; "Valve 2 Position" min=1 max=8; "Valve 1 Position" min=1 max=8; "Ramp Duration (s)" min=0.0 step=0.1; "Current End (pA)" step=0.1; "Replicates" min=1.0 step=1.0; "Current Start (pA)" step=0.1; "Ramp Slope (pA/s)" step=0.1; "Delay (s)" min=0.0 step=0.1; "Duration (s)" min=0.0 step=0.1}
  in  "Gap Free Iclamp J":T33={"Which Position to use for Experiment"=enum."Don't Move", "Duration (s)"=10.0, "Valve 1 Position"=2, "Valve 2 Position"=2, "Replicates"=5.0, "Iholding (pA)"=200.0, "Valve 3 Position"=2, "valve 1 used now?"=TRUE, "valve 2 used now?"=FALSE, "valve 3 used now? "=FALSE, "Record During Solution Change?"=FALSE} {"Valve 3 Position" min=1 max=8; "Iholding (pA)" step=0.1; "Replicates" min=1.0 step=1.0; "Valve 2 Position" min=1 max=8; "Valve 1 Position" min=1 max=8; "Duration (s)" min=0.0 step=0.1}
  in  "PhaseK Experiment Option":string(combo)="Single Manip Jump"
  in  "Experiment Selection K":T20(tab)=enum."Paired Pulse"
  in  "Single Jump K":T21={"Which Position to use for Experiment"=enum."Jumper Position B-A", "Start Position (N)"="Jumper Posistion B", "Jump Position (m)"="Jumper Posistion A", "Duration (s)"=5.0, "Delay (s)"=1.0, "Pulse Width (s)"=1.0, "Valve 1 Position"=2, "Valve 2 Position"=2, "Replicates"=10.0, "Vholding (mV)"=-60.0, "Valve 3 Position"=2, "valve 1 used now?"=TRUE, "valve 2 used now?"=FALSE, "valve 3 used now? "=FALSE, "protocol Preview"=[]} {"Valve 3 Position" min=1 max=8; "Vholding (mV)" step=0.1; "Replicates" min=1.0 step=1.0; "Valve 2 Position" min=1 max=8; "Valve 1 Position" min=1 max=8; "Pulse Width (s)" min=0.0 step=0.1; "Delay (s)" min=0.0 step=0.1; "Duration (s)" min=0.0 step=0.1}
  in  "Solution Change K":T22={"Which Position to use for Experiment"=enum."Jumper Safe Position", "Duration (s)"=60.0, "Delay (s)"=1.0, "Pulse Width (s)"=30.0, "Which Valve to Change?"=1, "Valve Jump Position"=3, "Replicates"=1.0, "Vholding (mV)"=-70.0, "valve 1 used now?"=TRUE, "valve 2 used now?"=FALSE, "valve 3 used now? "=FALSE, "Valve 1 Position"=2, "Valve 2 Position"=2, "Valve 3 Position"=2, "protocol Preview"=[]} {"Valve 3 Position" min=1 max=8; "Valve 2 Position" min=1 max=8; "Valve 1 Position" min=1 max=8; "Vholding (mV)" step=0.1; "Replicates" min=1.0 step=1.0; "Valve Jump Position" min=1 max=8 step=1; "Which Valve to Change?" min=1 max=8 step=1; "Pulse Width (s)" min=0.0 step=0.1; "Delay (s)" min=0.0 step=0.1; "Duration (s)" min=0.0 step=0.1}
  in  "Voltage Step K":T23={"Which Position to use for Experiment"=enum."Jumper Safe Position", "Duration (s)"=10.0, "Delay (s)"=1.0, "Step Width (s)"=0.1, "Voltage Start (mV)"=-60.0, "Voltage Step (mV)"=0.0, "Replicates"=1.0, "Voltage End (mV)"=40.0, "Number of Step"=20.0, "Vholding (mV)"=-60.0, "Valve 1 Position"=2, "Valve 2 Position"=2, "Valve 3 Position"=2, "valve 1 used now?"=TRUE, "valve 2 used now?"=FALSE, "valve 3 used now? "=FALSE, "Total Step Time (s)"=0.0, "Maintain Final Voltage until end?"=TRUE, "protocol Preview"=[]} {"Total Step Time (s)" min=0.0 step=0.1; "Valve 3 Position" min=1 max=8; "Valve 2 Position" min=1 max=8; "Valve 1 Position" min=1 max=8; "Vholding (mV)" step=0.1; "Number of Step" min=0.0 step=1.0; "Voltage End (mV)" step=0.1; "Replicates" min=1.0 step=1.0; "Voltage Step (mV)" step=0.1; "Voltage Start (mV)" step=0.1; "Step Width (s)" step=0.1; "Delay (s)" min=0.0 step=0.1; "Duration (s)" min=0.0 step=0.1}